vi "TLB Native Dynamic Events ver 0.25.vi"() -> ()   [LabVIEW 2018] (continued)
      tunnel: w233 -> [w2769 w2780 w2794 w2817 w2826 w2840 w2853 w2867 w2881 w2895 w2908 w2919 w2934 w2945 w2967 w2988 w3004 w3012 w3029 w3053 w3063 w3075 w3089 w3101 w3115 w3136 w3171 w3199 w3210 w3222 w3233 w3248 w3263 w3275 w3285 w3311 w3322 w3329 w3339 w3349 w3361 w3373 w3391 w3401 w3417 w3423 w3443 w3457 w3471 w3485 w3499 w3513 w3526]
      tunnel: [w2769 w2780 w2794 w2817 w2826 w2840 w2853 w2867 w2881 w2895 w2908 w2919 w2934 w2945 w2966 w2988 w3004 w3012 w3028 w3053 w3063 w3075 w3089 w3101 w3115 w3135 w3170 w3199 w3210 w3222 w3233 w3248 w3263 w3275 w3285 w3311 w3322 w3329 w3339 w3349 w3361 w3373 w3391 w3401 w3417 w3423 w3443 w3457 w3471 w3485 w3499 w3513 w3526] -> w232
      tunnel: w230 -> [w2767 w2779 w2795 w2818 w2827 w2841 w2854 w2866 w2882 w2896 w2907 w2918 w2933 w2944 w2963 w2989 w3005 w3011 w3025 w3050 w3062 w3074 w3088 w3100 w3114 w3133 w3168 w3197 w3209 w3221 w3232 w3247 w3262 w3274 w3284 w3312 w3323 w3328 w3338 w3348 w3360 w3372 w3392 w3402 w3418 w3422 w3437 w3451 w3465 w3479 w3493 w3507 w3520]
      tunnel: [w2767 w2779 w2795 w2818 w2827 w2841 w2854 w2866 w2882 w2896 w2907 w2918 w2933 w2944 w2963 w2989 w3005 w3011 w3025 w3050 w3062 w3074 w3088 w3100 w3113 w3132 w3167 w3197 w3209 w3221 w3232 w3247 w3262 w3274 w3284 w3312 w3323 w3328 w3338 w3348 w3360 w3372 w3392 w3402 w3418 w3422 w3437 w3449 w3463 w3477 w3491 w3505 w3519] -> w229
      tunnel: w227 -> [_ _ _ _ _ _ _ _ _ _ _ _ _ _ _ _ _ _ _ _ _ _ _ _ _ _ _ _ _ _ _ _ _ _ _ _ _ _ _ _ _ _ _ _ w3409 _ _ _ _ _ _ _ _]
      tunnel: [w2766 w2778 w2789 w2808 w2821 w2835 w2849 w2862 w2877 w2890 w2904 w2917 w2927 w2943 w2960 w2980 w3006 w3010 w3022 w3049 w3061 w3073 w3087 w3097 w3107 w3126 w3159 w3196 w3208 w3220 w3237 w3241 w3256 w3271 w3282 w3296 w3315 w3334 w3337 w3347 w3359 w3371 w3383 w3403 w3407 w3421 w3436 w3446 w3460 w3474 w3488 w3502 w3516] -> w223
      tunnel: w224 -> [w2766 w2778 w2789 w2808 w2821 w2835 w2849 w2862 w2877 w2890 w2904 w2917 w2927 w2943 w2960 w2981 w3006 w3010 w3022 w3049 w3061 w3073 w3087 w3097 w3107 w3127 w3160 w3196 w3208 w3220 w3237 w3241 w3256 w3271 w3282 w3296 w3315 w3334 w3337 w3347 w3359 w3371 w3383 w3403 w3407 w3421 w3436 w3446 w3460 w3474 w3488 w3502 w3516]
      tunnel: w221 -> [_ _ _ _ _ _ _ _ w2876 _ _ _ _ _ _ _ _ _ _ _ _ _ _ _ _ _ _ _ _ _ _ _ _ _ _ _ _ _ _ _ _ _ _ _ _ _ _ _ _ _ _ _ _]
      tunnel: w219 -> [w2765 w2777 w2788 w2802 w2820 w2834 w2848 w2861 w2874 w2889 w2903 w2916 w2926 w2942 w2959 w2976 w2999 w3009 w3020 w3048 w3060 w3072 w3086 w3096 w3110 w3129 w3163 w3195 w3207 w3219 w3229 w3240 w3255 w3270 w3281 w3293 w3314 w3325 w3336 w3346 w3358 w3370 w3382 w3394 w3406 w3420 w3435 w3445 w3459 w3473 w3487 w3501 w3515]
      tunnel: [w2765 w2777 w2788 w2802 w2820 w2834 w2848 w2861 w2874 w2889 w2903 w2916 w2926 w2942 w2959 w2976 w2998 w3009 w3020 w3048 w3060 w3072 w3086 w3096 w3109 w3128 w3162 w3195 w3207 w3219 w3229 w3240 w3255 w3270 w3281 w3293 w3314 w3325 w3336 w3346 w3358 w3370 w3382 w3394 w3406 w3420 w3435 w3445 w3459 w3473 w3487 w3501 w3515] -> w218
      tunnel: [_ _ _ _ _ _ _ _ _ _ _ _ _ _ _ _ _ _ _ _ _ _ _ _ _ _ _ _ _ _ _ _ _ _ _ w3292 _ _ _ _ _ _ _ _ _ _ _ _ _ _ _ _ _] -> w216
      tunnel: w214 -> [w2764 w2776 w2787 w2801 w2819 w2833 w2847 w2860 w2873 w2888 w2902 w2915 w2925 w2941 w2958 w2975 w2990 w3008 w3018 w3047 w3059 w3071 w3085 w3095 w3111 w3130 w3164 w3194 w3206 w3218 w3228 w3239 w3254 w3269 w3280 w3291 w3313 w3324 w3335 w3345 w3357 w3369 w3381 w3393 w3405 w3419 w3434 w3444 w3458 w3472 w3486 w3500 w3514]
      tunnel: [w2764 w2776 w2787 w2801 w2819 w2833 w2847 w2860 w2873 w2888 w2902 w2915 w2925 w2941 w2958 w2975 w2990 w3008 w3018 w3047 w3059 w3071 w3085 w3095 w3111 w3130 w3164 w3194 w3206 w3218 w3228 w3239 w3254 w3269 w3280 w3291 w3313 w3324 w3335 w3345 w3357 w3369 w3381 w3393 w3405 w3419 w3434 w3444 w3458 w3472 w3486 w3500 w3514] -> w213
      frame "Exit" {
        # ">>State Logic  >>"
        # ">>> Time cluster >>>"
        # ">>> Yaw >>>"
        # ">>> Stepper position >>>"
        # ">>> Encoders >>>"
        # ">>> Object detection >>>"
        # ">>> Ultrasonic Sensors Detect >>>"
        n70 = call "Imaq Dispose"("All Images? (No)"=TRUE) -> ()  [unwired: 5 in, 1 out]
      }
      frame "----Movement States----" {
        # ">>State Logic  >>"
        # ">>> Time cluster >>>"
        # ">>> Yaw >>>"
        # ">>> Stepper position >>>"
        # ">>> Encoders >>>"
        # ">>> Object detection >>>"
        # ">>> Ultrasonic Sensors Detect >>>"
      }
      frame "FORWARD" {
        # ">>State Logic  >>"
        # ">>> Time cluster >>>"
        # ">>> Yaw >>>"
        # ">>> Stepper position >>>"
        # ">>> Encoders >>>"
        # ">>> Object detection >>>"
        # ">>> Ultrasonic Sensors Detect >>>"
        n71 = Unbundle By Name(w2794) -> ("Yaw"=w2790:dbl)
        n72 = call "MOTOR CONTROL WITH PID AE.vi"("Yaw"=w2790, "Speed"=50.0, "Direction"=MOTOR_CONTROL_WITH_PID_AE_DIRECTION_TYPE_DEF."y-axis movement", "AE Mode"=MOTOR_CONTROL_WITH_PID_AE_DATA_MODE_TYPE_DEF."Write to AE") -> ()  [unwired: 1 out]
      }
      frame "FORWARD - IR ASSIST" {
        # ">>State Logic  >>"
        # ">>> Time cluster >>>"
        # ">>> Yaw >>>"
        # ">>> Stepper position >>>"
        # ">>> Encoders >>>"
        # ">>> Object detection >>>"
        # ">>> Ultrasonic Sensors Detect >>>"
        n73 = Unbundle By Name(w2808) -> ("Left IR Sensor"=w2807:dbl)
        n74 = Subtract(x=w2807, y=15.0) -> (x-y=w2805:dbl)
        n75 = Multiply(x=w2805, y=0.25) -> (x*y=w2803:dbl)
        n76 = call "MOTOR CONTROL WITH PID AE.vi"("Yaw"=w2803, "Speed"=30.0, "Direction"=MOTOR_CONTROL_WITH_PID_AE_DIRECTION_TYPE_DEF."y-axis movement", "AE Mode"=MOTOR_CONTROL_WITH_PID_AE_DATA_MODE_TYPE_DEF."Write to AE") -> ()  [unwired: 1 out]
      }
      frame "LEFT" {
        # ">>State Logic  >>"
        # ">>> Time cluster >>>"
        # ">>> Yaw >>>"
        # ">>> Stepper position >>>"
        # ">>> Encoders >>>"
        # ">>> Object detection >>>"
        # ">>> Ultrasonic Sensors Detect >>>"
        n77 = Unbundle By Name(w2826) -> ("Yaw"=w2823:dbl)
        n78 = call "MOTOR CONTROL WITH PID AE.vi"("Yaw"=w2823, "Speed"=-20.0, "Direction"=MOTOR_CONTROL_WITH_PID_AE_DIRECTION_TYPE_DEF."x-axis movement", "AE Mode"=MOTOR_CONTROL_WITH_PID_AE_DATA_MODE_TYPE_DEF."Write to AE") -> ()  [unwired: 1 out]
      }
      frame "RIGHT" {
        # ">>> Time cluster >>>"
        # ">>> Yaw >>>"
        # ">>> Stepper position >>>"
        # ">>> Encoders >>>"
        # ">>> Object detection >>>"
        # ">>> Ultrasonic Sensors Detect >>>"
        n79 = Unbundle By Name(w2840) -> ("Yaw"=w2836:dbl)
        n80 = call "MOTOR CONTROL WITH PID AE.vi"("Yaw"=w2836, "Speed"=20.0, "Direction"=MOTOR_CONTROL_WITH_PID_AE_DIRECTION_TYPE_DEF."x-axis movement", "AE Mode"=MOTOR_CONTROL_WITH_PID_AE_DATA_MODE_TYPE_DEF."Write to AE") -> ()  [unwired: 1 out]
      }
      frame "R-ACW" {
        # ">>> IR Sensors >>>"
        # ">>> Time cluster >>>"
        # ">>> Yaw >>>"
        # ">>> Stepper position >>>"
        # ">>> Encoders >>>"
        # ">>> Object detection >>>"
        # ">>> Ultrasonic Sensors Detect >>>"
        n81 = call "MOTOR CONTROL WITH PID AE.vi"("Speed"=10.0, "Direction"=MOTOR_CONTROL_WITH_PID_AE_DIRECTION_TYPE_DEF."rotation", "AE Mode"=MOTOR_CONTROL_WITH_PID_AE_DATA_MODE_TYPE_DEF."Write to AE") -> ()  [unwired: 1 in, 1 out]
      }
      frame "R-CW" {
        (unwired) -0.2 ("Speed")
        # ">>> Time cluster >>>"
        # ">>> Yaw >>>"
        # ">>> Stepper position >>>"
        # ">>> Encoders >>>"
        # ">>> Object detection >>>"
        # ">>> Ultrasonic Sensors Detect >>>"
        n82 = call "MOTOR CONTROL WITH PID AE.vi"("Speed"=-10.0, "Direction"=MOTOR_CONTROL_WITH_PID_AE_DIRECTION_TYPE_DEF."rotation", "AE Mode"=MOTOR_CONTROL_WITH_PID_AE_DATA_MODE_TYPE_DEF."Write to AE") -> ()  [unwired: 1 in, 1 out]
      }
      frame "X AXIS - SLOW" {
        # ">>> Line Sensor Cluster>>>"
        # ">>> IR Sensors >>>"
        # ">>> Time cluster >>>"
        # ">>> Yaw >>>"
        # ">>> Stepper position >>>"
        # ">>> Encoders >>>"
        # ">>> Object detection >>>"
        # ">>> Ultrasonic Sensors Detect >>>"
        n83 = Unbundle By Name(w2876) -> ("xSpeed"=w2875:dbl)
        n84 = Unbundle By Name(w2881) -> ("Yaw"=w2878:dbl)
        n85 = call "MOTOR CONTROL WITH PID AE.vi"("Yaw"=w2878, "Speed"=w2875, "Direction"=MOTOR_CONTROL_WITH_PID_AE_DIRECTION_TYPE_DEF."x-axis movement", "AE Mode"=MOTOR_CONTROL_WITH_PID_AE_DATA_MODE_TYPE_DEF."Write to AE") -> ()  [unwired: 1 out]
      }
      frame "REVERSE" {
        # ">>> Time cluster >>>"
        # ">>> Yaw >>>"
        # ">>> Stepper position >>>"
        # ">>> Encoders >>>"
        # ">>> Object detection >>>"
        # ">>> Ultrasonic Sensors Detect >>>"
        n86 = Unbundle By Name(w2895) -> ("Yaw"=w2891:dbl)
        n87 = call "MOTOR CONTROL WITH PID AE.vi"("Yaw"=w2891, "Speed"=-50.0, "Direction"=MOTOR_CONTROL_WITH_PID_AE_DIRECTION_TYPE_DEF."y-axis movement", "AE Mode"=MOTOR_CONTROL_WITH_PID_AE_DATA_MODE_TYPE_DEF."Write to AE") -> ()  [unwired: 1 out]
      }
      frame "STOP" {
        n88 = Wait (ms)(milliseconds to wait=u32 100) -> ()  [unwired: 1 out]
        n89 = call "MOTOR CONTROL WITH PID AE.vi"("Direction"=MOTOR_CONTROL_WITH_PID_AE_DIRECTION_TYPE_DEF."stop", "AE Mode"=MOTOR_CONTROL_WITH_PID_AE_DATA_MODE_TYPE_DEF."Write to AE") -> ()  [unwired: 2 in, 1 out]
      }
      frame "----SENSOR READING---- " {
      }
      frame "READ ENCODERS" {
        # ">>> Time cluster >>>"
        # ">>> Yaw >>>"
        # ">>> Stepper position >>>"
        # ">>> Object detection >>>"
        # ">>> Current encoder distance >>>"
        # ">>> Ultrasonic Sensors Detect >>>"
        n90 = call "MOTOR CONTROL WITH PID AE.vi"("AE Mode"=MOTOR_CONTROL_WITH_PID_AE_DATA_MODE_TYPE_DEF."Read from AE") -> ("Speed & distance"=w2931:T13)  [unwired: 3 in]
        n91 = Unbundle By Name(w2931) -> ("xDistance"=w2930:dbl, "yDistance"=w2929:dbl, "wDistance"=w2928:dbl)
        n92 = Bundle By Name(cluster=w2938, "xDistance"=w2930, "yDistance"=w2929, "wDistance"=w2928) -> (w2937:T6)
      }
      frame "READ ULTRASONIC" {
        (unwired) navX_type_def."Read Values" ("Mode")
        (unwired) MOTOR_CONTROL_NO_PID_Type_Def."Latch" ("Direction")
        # ">>> Line Sensor Cluster>>>"
        # ">>> IR Sensors >>>"
        # ">>State Logic  >>"
        # ">>> Time cluster >>>"
        # ">>> Ultrasonic Sensors Detect >>>"
        # ">>> Object detection >>>"
        # ">>> Encoders >>>"
        # ">>> Stepper position >>>"
        # ">>> Yaw >>>"
        n93 = call "Arduino Interfacing VI.vi"("AE Mode"=Arduino_Interfacing."Read From Arduino") -> ("Arduino Data"=w2950:T15)  [unwired: 3 in, 1 out]
        n94 = Unbundle By Name(w2950) -> ("PING A"=w2949:u8, "PING B"=w2948:u8, "PING C"=w2947:u8, "PING D"=w2946:u8)
        n95 = Bundle By Name(cluster=w2956, "PING_A"=w2949, "PING_B"=w2948, "PING_C"=w2947, "PING_D"=w2946) -> (w2957:T7)
      }
      frame "READ NAVX" {
        # ">> Item Selection Bias >>"
        # ">>State Logic  >>"
        # ">>> Line Sensor Cluster>>>"
        # ">>> IR Sensors >>>"
        # ">>> Time cluster >>>"
        # ">>> Yaw >>>"
        # ">>> Ultrasonic Sensors Detect >>>"
        # ">>> Object detection >>>"
        # ">>> Encoders >>>"
        # ">>> Stepper position >>>"
        n96 = call "navX reading VI.vi"("Mode"=navX_type_def."Read Values") -> ("NavX Readings"=w2962:T14)  [unwired: 2 in, 3 out]
        n97 = Unbundle By Name(w2962) -> ("Heading"=w2961:dbl)
        n98 = Unbundle By Name(w2962) -> ("Yaw"=w2965:dbl)
        n99 = Bundle By Name(cluster=w2967, "Yaw"=w2965, "Compass"=w2961) -> (w2966:T4)
      }
      frame "READ IR" {
        w2974 = T38 [enum."B/AI2"] items=["Not Connected", "AudioIn/Left", "AudioIn/Right", "C/AI0", "C/AI1", "A/AI0", "A/AI1", "A/AI2", "A/AI3", "A/AI4", "A/AI5", "A/AI6", "A/AI7", "B/AI0", "B/AI1", "B/AI2", "B/AI3", "B/AI4", "B/AI5", "B/AI6", "B/AI7", "AI/AI0", "AI/AI1", "AI/AI2", "AI/AI3", "A/AI0 (DIFF)", "A/AI1 (DIFF)", "A/AI2 (DIFF)", "A/AI3 (DIFF)", "B/AI0 (DIFF)", "B/AI1 (DIFF)", "B/AI2 (DIFF)", "B/AI3 (DIFF)"] ("AI Channel")
        w2978 = T38 [enum."B/AI1"] items=["Not Connected", "AudioIn/Left", "AudioIn/Right", "C/AI0", "C/AI1", "A/AI0", "A/AI1", "A/AI2", "A/AI3", "A/AI4", "A/AI5", "A/AI6", "A/AI7", "B/AI0", "B/AI1", "B/AI2", "B/AI3", "B/AI4", "B/AI5", "B/AI6", "B/AI7", "AI/AI0", "AI/AI1", "AI/AI2", "AI/AI3", "A/AI0 (DIFF)", "A/AI1 (DIFF)", "A/AI2 (DIFF)", "A/AI3 (DIFF)", "B/AI0 (DIFF)", "B/AI1 (DIFF)", "B/AI2 (DIFF)", "B/AI3 (DIFF)"] ("AI Channel")
        w2983 = T38 [enum."B/AI0"] items=["Not Connected", "AudioIn/Left", "AudioIn/Right", "C/AI0", "C/AI1", "A/AI0", "A/AI1", "A/AI2", "A/AI3", "A/AI4", "A/AI5", "A/AI6", "A/AI7", "B/AI0", "B/AI1", "B/AI2", "B/AI3", "B/AI4", "B/AI5", "B/AI6", "B/AI7", "AI/AI0", "AI/AI1", "AI/AI2", "AI/AI3", "A/AI0 (DIFF)", "A/AI1 (DIFF)", "A/AI2 (DIFF)", "A/AI3 (DIFF)", "B/AI0 (DIFF)", "B/AI1 (DIFF)", "B/AI2 (DIFF)", "B/AI3 (DIFF)"] ("AI Channel")
        # ">>> Line Sensor Cluster>>>"
        # ">>> IR Sensors >>>"
        # ">>State Logic  >>"
        # ">>> Time cluster >>>"
        # ">>> Ultrasonic Sensors Detect >>>"
        # ">>> Object detection >>>"
        # ">>> Encoders >>>"
        # ">>> Stepper position >>>"
        # ">>> Yaw >>>"
        n100 = call <vilib>:"Sharp IR.vi"("AI Channel"=w2983) -> ("Sharp IR Distance"=w2979:dbl)  [unwired: 8 in, 2 out]
        n101 = call <vilib>:"Sharp IR.vi"("AI Channel"=w2978) -> ("Sharp IR Distance"=w2977:dbl)  [unwired: 8 in, 2 out]
        n102 = call <vilib>:"Sharp IR.vi"("AI Channel"=w2974) -> ("Sharp IR Distance"=w2973:dbl)  [unwired: 8 in, 2 out]
        n103 = Bundle By Name(cluster=w2981, "Left IR Sensor"=w2979, "Arm IR Sensor"=w2977, "Bottom IR Sensor"=w2973) -> (w2980:T3)
      }
      frame "READ LINE SENSOR" {
        # ">>> IR Sensors >>>"
        # ">>> Line Sensor Cluster>>>"
        # ">>State Logic  >>"
        # ">>> Time cluster >>>"
        # ">>> Object detection >>>"
        # ">>> Yaw >>>"
        # ">>> Ultrasonic Sensors Detect >>>"
        # ">>> Encoders >>>"
        # ">>> Stepper position >>>"
        n104 = call "Line Sensor AE.vi"("AE State"=Line_Sensor_AE_Type_Def."READ FROM LINE SENSORS") -> ("Line Detected?"=w2996:bool, "Line Sensor Raw Values"=w2995:T40)
        n105 = Unbundle By Name(w2995) -> ("S1"=w2994:dbl, "S2"=w2993:dbl, "S3"=w2992:dbl, "S4"=w2991:dbl)
        n106 = Bundle By Name(cluster=w2999, "Line Detected?"=w2996, "S1"=w2994, "S2"=w2993, "S3"=w2992, "S4"=w2991) -> (w2998:T2)
      }
      frame "----SYSTEM MODES----" {
        (unwired) I2C_MASTER_Type_Def."Last State" ("Arduino Mode")
        # ">>> Object detection >>>"
        # ">>> Yaw >>>"
        # ">>> Ultrasonic Sensors Detect >>>"
        # ">>> Encoders >>>"
        # ">>> Stepper position >>>"
      }
      frame "INIT" {
        w3040 = u8 0
        w3041 = 0.0
        # ">>> IR Sensors >>>"
        # ">>> IR Sensors >>>"
        # ">>> Line Sensor Cluster>>>"
        # ">>> Time cluster >>>"
        # ">>> Object detection >>>"
        # ">>> Yaw >>>"
        # ">>> Ultrasonic Sensors Detect >>>"
        # ">>> Encoders >>>"
        # ">>> Stepper position >>>"
        # ">>State Logic  >>"
        n107 = call "Arduino Interfacing VI.vi"("AE Mode"=Arduino_Interfacing."Initialize") -> ()  [unwired: 3 in, 2 out]
        n108 = call "FGV Stop.vi"("Init/Read/Write State"=States_for_Action_Engine."Initialize") -> ()  [unwired: 2 in, 2 out]
        n109 = call "Elasped Timer.vi"("Action"=Elapsed_timer_control."Initialize") -> ()  [unwired: 7 in, 4 out]
        n110 = call "MOTOR CONTROL WITH PID AE.vi"("AE Mode"=MOTOR_CONTROL_WITH_PID_AE_DATA_MODE_TYPE_DEF."Init AE") -> ()  [unwired: 3 in, 1 out]
        n111 = call "IMAQ Reference AE.vi"("IMAQ AE States"=IMAQ_Reference_AE."Initialize AE") -> ()  [unwired: 1 in, 2 out]
        n112 = call "Line Sensor AE.vi"("AE State"=Line_Sensor_AE_Type_Def."INIT AE") -> ()  [unwired: 2 out]
        n113 = Bundle By Name(cluster=w3034, "Recognized Object"=FALSE, "Object X coordinate"=0.0, "Object Y coordinate"=0.0) -> (w3033:T9)
        n114 = Bundle By Name(cluster=w3039, "y Stepper Position"=u8 0, "z Stepper Position"=u8 0) -> (w3038:T5)
        n115 = Bundle By Name(cluster=w3043, "xDistance"=w3041, "yDistance"=w3041, "wDistance"=w3041) -> (w3042:T6)
        n116 = Bundle By Name(cluster=w3045, "PING_A"=w3040, "PING_B"=w3040, "PING_C"=w3040, "PING_D"=w3040) -> (w3046:T7)
        n117 = Bundle By Name(cluster=w3029, "Yaw"=0.0) -> (w3028:T4)
      }
      frame "ARDUINO - ULTRASONIC" {
        # ">>> Time cluster >>>"
        # ">>> Line Sensor Cluster>>>"
        # ">>> Object detection >>>"
        # ">>> Yaw >>>"
        # ">>> Ultrasonic Sensors Detect >>>"
        # ">>> Encoders >>>"
        # ">>> Stepper position >>>"
        # ">>State Logic  >>"
        n118 = call "Arduino Interfacing VI.vi"("Data to Write"=I2C_MASTER_WRITE_NEW_Type_Def."Ultrasonic sensors", "AE Mode"=Arduino_Interfacing."Write to Arduino") -> ()  [unwired: 2 in, 2 out]
      }
      frame "NAVX CALIBRATE" {
        # ">>> Object detection >>>"
        # ">>> Yaw >>>"
        # ">>> Ultrasonic Sensors Detect >>>"
        # ">>> Encoders >>>"
        # ">>> Stepper position >>>"
        # ">>State Logic  >>"
        # "Adds a 15 second delay to the startup process \nfor the NavX to calibrate"
        n119 = Wait (ms)(milliseconds to wait=u32 1000) -> ()  [unwired: 1 out]
      }
      frame "NO ACTION", Default {
        (unwired) u8 0 ("y Stepper value")
        (unwired) TRUE ("Latch")
        (unwired) navX_type_def."Read Values" ("Mode")
        (unwired) MOTOR_CONTROL_NO_PID_Type_Def."Latch" ("Direction")
        # ">>> Object detection >>>"
        # ">>> Yaw >>>"
        # ">>> Ultrasonic Sensors Detect >>>"
        # ">>> Encoders >>>"
        # ">>> Stepper position >>>"
        # ">>State Logic  >>"
        n120 = case shown="4" w3079 {
          tunnel: [0 100] -> w3081
          frame 1, Default {
          }
          frame 4 {
          }
        }
      }
      frame "----RESET CASES----" {
        (unwired) I2C_MASTER_Type_Def."Last State" ("Arduino Mode")
        # ">>> Object detection >>>"
        # ">>> Yaw >>>"
        # ">>> Ultrasonic Sensors Detect >>>"
        # ">>> Encoders >>>"
        # ">>> Stepper position >>>"
        # ">>State Logic  >>"
      }
      frame "RESET ENCODERS" {
        # ">>> Object detection >>>"
        # ">>> Yaw >>>"
        # ">>> Ultrasonic Sensors Detect >>>"
        # ">>> Encoders >>>"
        # ">>> Stepper position >>>"
        # ">>State Logic  >>"
        n121 = call "MOTOR CONTROL WITH PID AE.vi"("Direction"=MOTOR_CONTROL_WITH_PID_AE_DIRECTION_TYPE_DEF."reset encoders", "AE Mode"=MOTOR_CONTROL_WITH_PID_AE_DATA_MODE_TYPE_DEF."Write to AE") -> ()  [unwired: 2 in, 1 out]
      }
      frame "RESET FLAGS" {
        # ">>> Line Sensor Cluster>>>"
        # ">>> IR Sensors >>>"
        # ">>> Time cluster >>>"
        # ">>> Object detection >>>"
        # ">>> Yaw >>>"
        # ">>> Ultrasonic Sensors Detect >>>"
        # ">>> Encoders >>>"
        # ">>> Stepper position >>>"
        # ">>> Line Sensor Cluster>>>"
        # ">>> IR Sensors >>>"
        # ">>> Time cluster >>>"
        # ">>> Object detection >>>"
        # ">>> Yaw >>>"
        # ">>> Ultrasonic Sensors Detect >>>"
        # ">>> Encoders >>>"
        # ">>> Stepper position >>>"
        # "Resets BOOLEAN FLAGS only"
        n122 = Wait (ms)(milliseconds to wait=u32 20) -> ()  [unwired: 1 out]
        n123 = Bundle By Name(cluster=w3120, "Recognized Object"=FALSE) -> (w3119:T9)
        n124 = Bundle By Name(cluster=w3110, "Line Detected?"=FALSE) -> (w3109:T2)
        n125 = Bundle By Name(cluster=w3114, "Time up flag"=FALSE) -> (w3113:T1)
      }
      frame "RESET SENSOR VALUES" {
        w3124 = 0.0 ("S4")
        w3125 = 0.0 ("S4")
        # "Resets SENSOR VALUES only"
        # ">>> Line Sensor Cluster>>>"
        # ">>> IR Sensors >>>"
        # ">>> Time cluster >>>"
        # ">>> Object detection >>>"
        # ">>> Yaw >>>"
        # ">>> Ultrasonic Sensors Detect >>>"
        # ">>> Encoders >>>"
        # ">>> Stepper position >>>"
        # ">>> Line Sensor Cluster>>>"
        # ">>> IR Sensors >>>"
        # ">>> Time cluster >>>"
        # ">>> Object detection >>>"
        # ">>> Yaw >>>"
        # ">>> Ultrasonic Sensors Detect >>>"
        # ">>> Encoders >>>"
        # ">>> Stepper position >>>"
        # "Resets any software variables\nand/or non-critical states"
        n126 = Wait (ms)(milliseconds to wait=u32 20) -> ()  [unwired: 1 out]
        n127 = Bundle By Name(cluster=w3133, "SET TIME TO CHECK"=0.0) -> (w3132:T1)
        n128 = Bundle By Name(cluster=w3149, "Object X coordinate"=0.0, "Object Y coordinate"=0.0) -> (w3148:T9)
        n129 = Bundle By Name(cluster=w3140, "y Stepper Position"=u8 0, "z Stepper Position"=u8 0) -> (w3139:T5)
        n130 = Bundle By Name(cluster=w3127, "Left IR Sensor"=w3124, "Arm IR Sensor"=w3124) -> (w3126:T3)
        n131 = Bundle By Name(cluster=w3145, "xDistance"=0.0, "yDistance"=0.0, "wDistance"=0.0) -> (w3144:T6)
        n132 = Bundle By Name(cluster=w3156, "PING_A"=u8 0, "PING_B"=u8 0, "PING_C"=u8 0, "PING_D"=u8 0) -> (w3155:T7)
        n133 = Bundle By Name(cluster=w3136, "Yaw"=0.0) -> (w3135:T4)
        n134 = Bundle By Name(cluster=w3129, "S1"=w3125, "S2"=w3125, "S3"=w3125, "S4"=w3125) -> (w3128:T2)
      }
      frame "RESET ALL SENSORS" {
        w3158 = 0.0 ("SET TIME TO CHECK")
        # ">>> Line Sensor Cluster>>>"
        # ">>> IR Sensors >>>"
        # ">>> Time cluster >>>"
        # ">>> Object detection >>>"
        # ">>> Yaw >>>"
        # ">>> Ultrasonic Sensors Detect >>>"
        # ">>> Encoders >>>"
        # ">>> Stepper position >>>"
        # ">>> Line Sensor Cluster>>>"
        # ">>> IR Sensors >>>"
        # ">>> Time cluster >>>"
        # ">>> Object detection >>>"
        # ">>> Yaw >>>"
        # ">>> Ultrasonic Sensors Detect >>>"
        # ">>> Encoders >>>"
        # ">>> Stepper position >>>"
        # "Resets ALL SENSOR PARAMTERS"
        n135 = Wait (ms)(milliseconds to wait=u32 20) -> ()  [unwired: 1 out]
        n136 = Bundle By Name(cluster=w3168, "Time up flag"=FALSE, "SET TIME TO CHECK"=0.0) -> (w3167:T1)
        n137 = Bundle By Name(cluster=w3185, "Recognized Object"=FALSE, "Object X coordinate"=0.0, "Object Y coordinate"=0.0) -> (w3184:T9)
        n138 = Bundle By Name(cluster=w3175, "y Stepper Position"=u8 0, "z Stepper Position"=u8 0) -> (w3174:T5)
        n139 = Bundle By Name(cluster=w3163, "Line Detected?"=FALSE) -> (w3162:T2)
        n140 = Bundle By Name(cluster=w3160, "Left IR Sensor"=w3158, "Arm IR Sensor"=w3158) -> (w3159:T3)
        n141 = Bundle By Name(cluster=w3180, "xDistance"=0.0, "yDistance"=0.0, "wDistance"=0.0) -> (w3179:T6)
        n142 = Bundle By Name(cluster=w3192, "PING_A"=u8 0, "PING_B"=u8 0, "PING_C"=u8 0, "PING_D"=u8 0) -> (w3191:T7)
        n143 = Bundle By Name(cluster=w3171, "Yaw"=0.0) -> (w3170:T4)
      }
      frame "RESET YAW" {
        n144 = Wait (ms)(milliseconds to wait=u32 100) -> ()  [unwired: 1 out]
        n145 = call "navX reading VI.vi"("Mode"=navX_type_def."Zero Yaw") -> ()  [unwired: 2 in, 4 out]
      }
      frame "RESET ARM" {
        n146 = call "Arduino Interfacing VI.vi"("Data to Write"=I2C_MASTER_WRITE_NEW_Type_Def."Soft Reset", "AE Mode"=Arduino_Interfacing."Write to Arduino") -> ()  [unwired: 2 in, 2 out]
      }
      frame "--------CAM STATES-------" {
      }
      frame "OPEN IMAQ REF" {
        # ">>> Line Sensor Cluster>>>"
        # ">>State Logic  >>"
        # ">>> Time cluster >>>"
        # ">>> Object detection >>>"
        # ">>> Yaw >>>"
        # ">>> Ultrasonic Sensors Detect >>>"
        # ">>> Encoders >>>"
        # ">>> Stepper position >>>"
        # ">>> IR Sensors >>>"
        n147 = call "IMAQ Reference AE.vi"("IMAQ AE States"=IMAQ_Reference_AE."Initialize AE") -> ()  [unwired: 1 in, 2 out]
      }
      frame "OPEN LOG CAM" {
        n148 = call "Webcam AE.vi"("Session In"=T36 "cam0", "Camera states"=Webcam_AE."Initialize Camera") -> ("error out"=w3244:errorcluster, "Session Out"=w3243:T36)  [unwired: 1 in, 1 out]
        n149 = call "Webcam AE.vi"("error in (no error)"=w3244, "Session In"=w3243, "Camera states"=Webcam_AE."Open Camera") -> ()  [unwired: 3 out]
      }
      frame "OPEN LIFE CAM" {
        n150 = call "Webcam AE.vi"("Session In"=T36 "cam1", "Camera states"=Webcam_AE."Initialize Camera") -> ("error out"=w3259:errorcluster, "Session Out"=w3258:T36)  [unwired: 1 in, 1 out]
        n151 = call "Webcam AE.vi"("error in (no error)"=w3259, "Session In"=w3258, "Camera states"=Webcam_AE."Open Camera") -> ()  [unwired: 3 out]
      }
      frame "CAM ACQ" {
        # ">>State Logic  >>"
        # ">>> Time cluster >>>"
        # ">>> Yaw >>>"
        # ">>> Stepper position >>>"
        # ">>> Encoders >>>"
        # ">>> Object detection >>>"
        # ">>> Ultrasonic Sensors Detect >>>"
        n152 = call "Webcam AE.vi"("Camera states"=Webcam_AE."Continuous Acquisition") -> ()  [unwired: 2 in, 3 out]
      }
      frame "CAM CLOSE" {
        # ">>State Logic  >>"
        # ">>> Time cluster >>>"
        # ">>> Yaw >>>"
        # ">>> Stepper position >>>"
        # ">>> Encoders >>>"
        # ">>> Object detection >>>"
        # ">>> Ultrasonic Sensors Detect >>>"
        n153 = call "Webcam AE.vi"("Camera states"=Webcam_AE."Close Camera") -> ()  [unwired: 2 in, 3 out]
      }
      frame "PROCESS IMAGE" {
        # ">>> Line Sensor Cluster>>>"
        # ">>> IR Sensors >>>"
        # ">> Item Selection Bias >>"
        # ">> Item Selection Bias >>"
        # ">>State Logic  >>"
        # ">>> Time cluster >>>"
        # ">>> Yaw >>>"
        # ">>> Stepper position >>>"
        # ">>> Encoders >>>"
        # ">>> Object detection >>>"
        # ">>> Ultrasonic Sensors Detect >>>"
        n154 = call "Webcam AE.vi"("Camera states"=Webcam_AE."Retrieve Image") -> ("error out"=w3304:errorcluster, "Image Out"=w3305:T42)  [unwired: 2 in, 1 out]
        n155 = call "IMAQ Reference AE.vi"("IMAQ AE States"=IMAQ_Reference_AE."Get IMAQ Reference") -> ("Image Out"=w3294:T42)  [unwired: 1 in, 1 out]
        n156 = call "Object Detection SubVI.vi"("Error In"=w3304, "Mode"=w3291, "Image Dest"=w3294, "Image in"=w3305) -> ("Error out"=w3292:errorcluster, "Object Center Coordinates"=w3301:cluster{"x":sgl, "y":sgl}, "Object detection cluster"=w3297:T43)  [unwired: 1 out]
        n157 = Unbundle By Name(w3297) -> ("Object detected?"=w3298:bool)
        n158 = Unbundle By Name(w3301) -> ("x"=w3300:sgl, "y"=w3299:sgl)
        n159 = Bundle By Name(cluster=w3303, "Recognized Object"=w3298, "Object X coordinate"=w3300, "Object Y coordinate"=w3299) -> (w3302:T9)
      }
      frame "DISPOSE CAM BUFFERS" {
        # ">> Item Selection Bias >>"
        # ">>> Line Sensor Cluster>>>"
        # ">>> IR Sensors >>>"
        # ">>State Logic  >>"
        # ">>> Time cluster >>>"
        # ">>> Yaw >>>"
        # ">>> Stepper position >>>"
        # ">>> Encoders >>>"
        # ">>> Object detection >>>"
        # ">>> Ultrasonic Sensors Detect >>>"
        n160 = call "Webcam AE.vi"("Camera states"=Webcam_AE."Dispose Camera Image Buffer") -> ()  [unwired: 2 in, 3 out]
      }
      frame "DISPOSE PROC BUFFERS" {
        # ">>> Line Sensor Cluster>>>"
        # ">>State Logic  >>"
        # ">>> IR Sensors >>>"
        # ">>> Time cluster >>>"
        # ">>> Object detection >>>"
        # ">>> Yaw >>>"
        # ">>> Ultrasonic Sensors Detect >>>"
        # ">>> Encoders >>>"
        # ">>> Stepper position >>>"
        n161 = call "IMAQ Reference AE.vi"("IMAQ AE States"=IMAQ_Reference_AE."Dispose Processing Buffer") -> ()  [unwired: 1 in, 2 out]
      }
      frame "-----ARM ACTIONS-----" {
      }
      frame "CLOSE CLAW" {
        n162 = call "Arduino Interfacing VI.vi"("Data to Write"=I2C_MASTER_WRITE_NEW_Type_Def."Close Claw", "AE Mode"=Arduino_Interfacing."Write to Arduino") -> ()  [unwired: 2 in, 2 out]
      }
      frame "OPEN CLAW" {
        n163 = call "Arduino Interfacing VI.vi"("Data to Write"=I2C_MASTER_WRITE_NEW_Type_Def."Open Claw", "AE Mode"=Arduino_Interfacing."Write to Arduino") -> ()  [unwired: 2 in, 2 out]
      }
      frame "Z STEPPER CAM HEIGHT" {
        n164 = call "Arduino Interfacing VI.vi"("Data to Write"=I2C_MASTER_WRITE_NEW_Type_Def."zStepper 6k", "AE Mode"=Arduino_Interfacing."Write to Arduino") -> ()  [unwired: 2 in, 2 out]
      }
      frame "Z STEPPER GRAB HEIGHT" {
        # ">>State Logic  >>"
        # ">>> Time cluster >>>"
        # ">>> Yaw >>>"
        # ">>> Stepper position >>>"
        # ">>> Encoders >>>"
        # ">>> Object detection >>>"
        # ">>> Ultrasonic Sensors Detect >>>"
        n165 = call "Arduino Interfacing VI.vi"("Data to Write"=I2C_MASTER_WRITE_NEW_Type_Def."zStepper 100", "AE Mode"=Arduino_Interfacing."Write to Arduino") -> ()  [unwired: 2 in, 2 out]
      }
      frame "Z STEPPER BOX HEIGHT" {
        # ">>> IR Sensors >>>"
        # ">>> Time cluster >>>"
        # ">>> Yaw >>>"
        # ">>> Stepper position >>>"
        # ">>> Encoders >>>"
        # ">>> Object detection >>>"
        # ">>> Ultrasonic Sensors Detect >>>"
        n166 = call "Arduino Interfacing VI.vi"("Data to Write"=I2C_MASTER_WRITE_NEW_Type_Def."zStepper 4k", "AE Mode"=Arduino_Interfacing."Write to Arduino") -> ()  [unwired: 2 in, 2 out]
      }
      frame "Y STEPPER CONTROL" {
        # ">>State Logic  >>"
        # ">>> yStepper command>>>"
        # ">>> Time cluster >>>"
        # ">>> Yaw >>>"
        # ">>> Stepper position >>>"
        # ">>> Encoders >>>"
        # ">>> Object detection >>>"
        # ">>> Ultrasonic Sensors Detect >>>"
        n167 = Unbundle By Name(w3409) -> ("yStepper desired"=w3408:u8)
        n168 = call "Arduino Interfacing VI.vi"("y Stepper value"=w3408, "Data to Write"=I2C_MASTER_WRITE_NEW_Type_Def."yStepper control", "AE Mode"=Arduino_Interfacing."Write to Arduino") -> ()  [unwired: 1 in, 2 out]
      }
      frame "READ STEPPER VALUES" {
        # ">>State Logic  >>"
        # ">>> Time cluster >>>"
        # ">>> Yaw >>>"
        # ">>> Stepper position >>>"
        # ">>> Encoders >>>"
        # ">>> Object detection >>>"
        # ">>> Ultrasonic Sensors Detect >>>"
        n169 = call "Arduino Interfacing VI.vi"("AE Mode"=Arduino_Interfacing."Read From Arduino") -> ("Arduino Data"=w3426:T15)  [unwired: 3 in, 1 out]
        n170 = Unbundle By Name(w3426) -> ("y Stepper Position"=w3425:u8, "z Stepper Position"=w3424:u8)
        n171 = Bundle By Name(cluster=w3429, "y Stepper Position"=w3425, "z Stepper Position"=w3424) -> (w3428:T5)
      }
      frame " -----TIMING-----" {
        # ">>State Logic  >>"
        # ">>> Time cluster >>>"
        # ">>> Yaw >>>"
        # ">>> Stepper position >>>"
        # ">>> Encoders >>>"
        # ">>> Object detection >>>"
        # ">>> Ultrasonic Sensors Detect >>>"
      }
      frame "SET TIMER 1" {
        # ">>State Logic  >>"
        # ">>> Time cluster >>>"
        # ">>> Yaw >>>"
        # ">>> Stepper position >>>"
        # ">>> Encoders >>>"
        # ">>> Object detection >>>"
        # ">>> Ultrasonic Sensors Detect >>>"
        n172 = call "Elasped Timer.vi"("Time Setting"=1.0, "Action"=Elapsed_timer_control."Initialize") -> ()  [unwired: 6 in, 4 out]
        n173 = Bundle By Name(cluster=w3451, "Time up flag"=FALSE) -> (w3449:T1)
      }
      frame "SET TIMER 2" {
        # ">>State Logic  >>"
        # ">>> Time cluster >>>"
        # ">>> Yaw >>>"
        # ">>> Stepper position >>>"
        # ">>> Encoders >>>"
        # ">>> Object detection >>>"
        # ">>> Ultrasonic Sensors Detect >>>"
        n174 = call "Elasped Timer.vi"("Time Setting"=2.0, "Action"=Elapsed_timer_control."Initialize") -> ()  [unwired: 6 in, 4 out]
        n175 = Bundle By Name(cluster=w3465, "Time up flag"=FALSE) -> (w3463:T1)
      }
      frame "SET TIMER 3" {
        # ">>State Logic  >>"
        # ">>> Time cluster >>>"
        # ">>> Yaw >>>"
        # ">>> Stepper position >>>"
        # ">>> Encoders >>>"
        # ">>> Object detection >>>"
        # ">>> Ultrasonic Sensors Detect >>>"
        n176 = call "Elasped Timer.vi"("Time Setting"=3.0, "Action"=Elapsed_timer_control."Initialize") -> ()  [unwired: 6 in, 4 out]
        n177 = Bundle By Name(cluster=w3479, "Time up flag"=FALSE) -> (w3477:T1)
      }
      frame "SET TIMER 4" {
        # ">>State Logic  >>"
        # ">>> Time cluster >>>"
        # ">>> Yaw >>>"
        # ">>> Stepper position >>>"
        # ">>> Encoders >>>"
        # ">>> Object detection >>>"
        # ">>> Ultrasonic Sensors Detect >>>"
        n178 = call "Elasped Timer.vi"("Time Setting"=4.0, "Action"=Elapsed_timer_control."Initialize") -> ()  [unwired: 6 in, 4 out]
        n179 = Bundle By Name(cluster=w3493, "Time up flag"=FALSE) -> (w3491:T1)
      }
      frame "SET TIMER 5" {
        # ">>State Logic  >>"
        # ">>> Time cluster >>>"
        # ">>> Yaw >>>"
        # ">>> Stepper position >>>"
        # ">>> Encoders >>>"
        # ">>> Object detection >>>"
        # ">>> Ultrasonic Sensors Detect >>>"
        n180 = call "Elasped Timer.vi"("Time Setting"=5.0, "Action"=Elapsed_timer_control."Initialize") -> ()  [unwired: 6 in, 4 out]
        n181 = Bundle By Name(cluster=w3507, "Time up flag"=FALSE) -> (w3505:T1)
      }
      frame "START TIMER" {
        # ">>State Logic  >>"
        # ">>> Time cluster >>>"
        # ">>> Yaw >>>"
        # ">>> Stepper position >>>"
        # ">>> Encoders >>>"
        # ">>> Object detection >>>"
        # ">>> Ultrasonic Sensors Detect >>>"
        n182 = call "Elasped Timer.vi"("Action"=Elapsed_timer_control."Start") -> ("Time Out?!"=w3517:bool)  [unwired: 7 in, 3 out]
        n183 = Bundle By Name(cluster=w3520, "Time up flag"=w3517) -> (w3519:T1)
      }
    }
    "State Logic" <- w249
    "Image Processing Error" <- w216
    n184 = local read "TASK ENABLE"() -> (w243:bool)
    n185 = Not(x=w243) -> (.not. x?=w242:bool)
    n186 = case shown="True" w250 {
      tunnel: w254 -> [w281 w325]
      tunnel: w258 -> [w277 w327]
      tunnel: [w281 w325] -> w263
      tunnel: [w277 w328] -> w262
      tunnel: w259 -> [_ w323]
      tunnel: w261 -> [_ w324]
      tunnel: w256 -> [w280 w330]
      tunnel: [w280 w330] -> w255
      tunnel: "STOP TASK" -> [_ w313]
      tunnel: w249 -> [w279 w329]
      tunnel: [w279 w326] -> w248
      tunnel: w245 -> [w278 w319]
      tunnel: [w278 w319] -> w244
      tunnel: w242 -> [_ w314]
      tunnel: [w276 w311] -> w241
      tunnel: w240 -> [w276 w310]
      tunnel: w238 -> [w275 w307]
      tunnel: [w275 w307] -> w237
      tunnel: w235 -> [w274 w303]
      tunnel: [w274 w303] -> w234
      tunnel: w232 -> [w273 w301]
      tunnel: [w273 w301] -> w231
      tunnel: w229 -> [w272 w299]
      tunnel: [w272 w299] -> w228
      tunnel: w227 -> [w271 w298]
      tunnel: [w271 w297] -> w226
      tunnel: [_ w295] -> w225
      tunnel: w223 -> [w270 w293]
      tunnel: [w270 w293] -> w222
      tunnel: w221 -> [w269 w292]
      tunnel: [w269 w291] -> w220
      tunnel: w218 -> [w268 w288]
      tunnel: [w268 w288] -> w217
      tunnel: [w267 w287] -> w215
      tunnel: w213 -> [w267 w286]
      tunnel: [_ w284] -> w212
      tunnel: [_ w283] -> w211
      tunnel: [_ w282] -> w210
      frame False {
        # ">> Item Selection Bias >>"
        # ">>State Logic Queue Reference >>"
        # ">>Action states Queue Reference >>"
        # ">>True Stop Next State >>"
        # ">>State Logic  >>"
        # ">>> IR Sensors >>>"
        # ">>> Line Sensor Cluster>>>"
        # ">>> Line Sensor Cluster>>>"
        # ">>> Motor control cluster >>>"
        # ">>> yStepper command>>>"
        # ">>> Motor control cluster >>>"
        # ">>> yStepper command>>>"
        # ">>> Motor control cluster >>>"
        # ">>> IR Sensors >>>"
        # ">>> IR Sensors >>>"
        # ">>> yStepper command>>>"
        # ">>> Time cluster >>>"
        # ">>> Yaw >>>"
        # ">>> Stepper position >>>"
        # ">>> Encoders >>>"
        # ">>> Object detection >>>"
        # ">>> Ultrasonic Sensors Detect >>>"
        # ">>> Time cluster >>>"
        # ">>> Yaw >>>"
        # ">>> Stepper position >>>"
        # ">>> Encoders >>>"
        # ">>> Object detection >>>"
        # ">>> Ultrasonic Sensors Detect >>>"
      }
      frame True {
        # ">> Item Selection Bias >>"
        # ">>> IR Sensors >>>"
        # ">>> Line Sensor Cluster>>>"
        # ">>> Line Sensor Cluster>>>"
        # ">>> Motor control cluster >>>"
        # ">>> yStepper command>>>"
        # ">>> IR Sensors >>>"
        # ">>> Motor control cluster >>>"
        # ">>State Logic Queue Reference >>"
        # ">>Timeout>>"
        # ">>> yStepper command>>>"
        # ">>> Time cluster >>>"
        # ">>> Object detection >>>"
        # ">>> Yaw >>>"
        # ">>> Ultrasonic Sensors Detect >>>"
        # ">>> Encoders >>>"
        # ">>> Stepper position >>>"
        # ">>State Logic  >>"
        # ">>True Stop Next State >>"
        # ">>Action Queue>>"
        # ">> Manual override >>"
        # ">>> Time cluster >>>"
        # ">>> Yaw >>>"
        # ">>> Stepper position >>>"
        # ">>> Encoders >>>"
        # ">>> Object detection >>>"
        # ">>> Ultrasonic Sensors Detect >>>"
        # ">>Action Queue>>"
        # ">>State Logic Queue Reference >>"
        n187 = Or(x=w313, y=w314) -> (x .or. y?=w312:bool)
        n188 = Unbundle By Name(w293) -> ("Left IR Sensor"=w294:dbl, "Arm IR Sensor"=w290:dbl, "Bottom IR Sensor"=w285:dbl)
        n189 = Unbundle By Name(w288) -> ("Line Detected?"=w289:bool)
        n190 = Unbundle By Name(w299) -> ("Time up flag"=w300:bool)
        n191 = Unbundle By Name(w301) -> ("Yaw"=w302:dbl, "Compass"=w296:dbl)
        n192 = Unbundle By Name(w303) -> ("y Stepper Position"=w305:u8, "z Stepper Position"=w304:u8)
        n193 = Unbundle By Name(w319) -> ("xDistance"=w316:dbl, "yDistance"=w317:dbl, "wDistance"=w318:dbl)
        n194 = Unbundle By Name(w307) -> ("Recognized Object"=w306:bool, "Object X coordinate"=w309:dbl, "Object Y coordinate"=w308:dbl)
        n195 = Unbundle By Name(w330) -> ("PING_A"=w322:u8, "PING_B"=w321:u8, "PING_C"=w320:u8, "PING_D"=w315:u8)
        n196 = case shown="1" w329 {
          tunnel: [w335 w347 w361 w372 w490 w507 w553 w590 w645 w687 w735 w779 w834 w882 w926 w986 w1027 w1070 w1119 w1162 w1215 w1253 w1305 w1349 w1393 w1423 w1441 w1487 w1528 w1577 w1630 w1669 w1718 w1761 w1814 w1852 w1904 w1940 w1989 w2032 w2082 w2126 w2171 w2223 w2264 w2312 w2351 w2393 w2448 w2502 w2540 w2586 w2635 w2676 w2720] -> w328
          tunnel: w327 -> [w335 w350 w362 w375 w492 w508 w554 w599 w643 w691 w736 w785 w827 w885 w933 w976 w1030 w1076 w1118 w1165 w1205 w1259 w1295 w1344 w1384 w1423 w1431 w1490 w1534 w1576 w1629 w1675 w1717 w1764 w1804 w1858 w1894 w1944 w1996 w2037 w2087 w2131 w2175 w2221 w2265 w2313 w2353 w2403 w2458 w2501 w2544 w2592 w2634 w2680 w2724]
          tunnel: [State_Type_Definitions,_for_0.26g_versions_and_later_2."Idle" ("Enum") State_Type_Definitions,_for_0.26g_versions_and_later_2."Idle" ("Enum") w357 w374 State_Type_Definitions,_for_0.26g_versions_and_later_2."Shutdown" ("Enum") w509 w555 w597 w646 w688 w734 w780 w833 w883 w928 w985 w1028 w1077 w1120 w1164 w1214 w1260 w1304 w1350 w1385 State_Type_Definitions,_for_0.26g_versions_and_later_2."Idle" ("Enum") w1440 w1488 w1535 w1578 w1631 w1676 w1719 w1763 w1813 w1859 w1903 w1941 w1990 w2033 w2083 w2127 w2172 w2224 w2263 w2311 w2352 w2398 w2459 w2503 w2541 w2587 w2636 w2677 w2721] -> w326
          tunnel: w325 -> [_ _ w360 w378 _ w513 w560 w593 w642 w692 w743 w784 w831 w886 w932 w983 w1025 w1075 w1116 w1166 w1212 w1258 w1302 w1347 w1392 _ w1438 w1485 w1533 w1574 w1627 w1674 w1715 w1765 w1811 w1857 w1901 w1948 w1995 w2040 w2090 w2134 w2178 w2220 w2266 w2306 w2354 w2402 w2457 w2500 w2548 w2591 w2633 w2684 w2725]
          tunnel: w324 -> [_ _ _ w377 _ w512 w559 w592 w641 w693 w742 w783 w830 w879 w931 w982 w1024 w1074 w1115 w1167 w1211 w1257 w1301 w1346 w1390 _ w1437 w1484 w1532 w1573 w1626 w1673 w1714 w1766 w1810 w1856 w1900 w1943 w1994 w2039 w2089 w2133 w2174 w2219 w2267 w2307 w2355 w2401 w2456 w2499 w2547 w2590 w2632 w2683 w2726]
          tunnel: w323 -> [_ _ w359 w373 _ w511 w558 w591 w640 w694 w741 w782 w829 w878 w930 w984 w1026 w1073 w1114 w1168 w1213 w1256 w1303 w1345 w1391 _ w1439 w1486 w1531 w1572 w1625 w1672 w1713 w1767 w1812 w1855 w1902 w1947 w1993 w2038 w2088 w2132 w2177 w2218 w2268 w2308 w2356 w2400 w2455 w2498 w2546 w2589 w2631 w2682 w2727]
          tunnel: w312 -> [_ _ _ _ _ w498 w552 w598 w639 w695 w738 w778 w832 w884 w934 w977 w1031 w1071 w1117 w1169 w1206 w1254 w1296 w1348 w1388 _ w1432 w1491 w1529 w1575 w1628 w1670 w1716 w1768 w1805 w1853 w1895 w1946 w1988 w2036 w2086 w2130 w2176 w2217 w2269 w2309 w2357 w2399 w2454 w2497 w2545 w2588 w2630 w2681 w2728]
          tunnel: w322 -> [_ _ _ _ _ _ _ _ _ _ _ _ _ _ _ _ _ _ _ _ _ _ _ _ _ _ _ _ _ _ _ _ _ _ _ _ _ _ _ _ _ _ _ _ _ _ _ _ _ _ _ _ _ _ _]
          tunnel: w321 -> [_ _ _ _ _ _ _ _ w638 _ _ _ w823 w867 w924 _ _ _ _ _ _ _ _ _ _ _ _ w1477 _ _ _ _ _ _ _ _ _ _ _ _ _ _ _ _ _ _ _ _ w2452 _ _ _ _ _ _]
          tunnel: w320 -> [_ _ _ _ _ _ _ _ w637 _ _ _ w824 w868 w925 _ _ _ _ _ _ _ _ _ _ _ _ w1478 _ _ _ _ _ _ _ _ _ _ _ _ _ _ _ _ _ _ _ _ w2453 _ _ _ _ _ _]
          tunnel: w318 -> [_ _ _ _ _ _ _ _ _ _ w740 _ _ _ _ _ _ _ _ _ _ _ _ _ _ _ _ _ _ _ _ _ _ _ _ _ _ _ _ _ _ _ _ _ _ _ _ w2396 _ _ _ _ _ _ _]
          tunnel: w317 -> [_ _ _ _ _ w506 w551 _ _ w686 _ _ _ _ w929 _ _ _ _ _ _ _ _ _ _ _ _ _ _ _ _ _ _ _ _ _ _ _ _ _ _ _ _ _ _ _ _ _ w2444 _ _ _ _ _ _]
          tunnel: w316 -> [_ _ _ _ _ _ _ _ _ _ _ _ _ w873 _ _ _ _ _ _ _ _ _ _ _ _ _ _ _ _ w1616 _ _ _ _ _ _ _ _ _ _ _ _ _ w2258 _ _ _ _ _ _ _ w2629 _ _]
          tunnel: w315 -> [_ _ _ _ _ _ _ _ _ _ _ _ _ _ _ _ _ _ _ _ _ _ _ _ _ _ _ _ _ _ _ _ _ _ _ _ _ _ _ _ _ _ _ _ _ _ _ _ _ _ _ _ _ _ _]
          tunnel: [State_Type_Definitions,_for_0.26g_versions_and_later_2."Idle" ("Enum") State_Type_Definitions,_for_0.26g_versions_and_later_2."Idle" ("Enum") State_Type_Definitions,_for_0.26g_versions_and_later_2."Idle" ("Enum") State_Type_Definitions,_for_0.26g_versions_and_later_2."Idle" ("Enum") State_Type_Definitions,_for_0.26g_versions_and_later_2."Shutdown" ("Enum") w504 w549 w596 w644 w689 w731 w777 w826 w881 w927 w987 w1029 w1069 w1121 w1163 w1216 w1252 w1306 w1351 w1386 w1425 w1442 w1489 w1527 w1579 w1632 w1668 w1720 w1762 w1815 w1851 w1905 w1942 w1991 w2035 w2085 w2129 w2173 w2222 w2262 w2310 w2350 w2397 w2460 w2504 w2542 w2585 w2637 w2678 w2722] -> w311
          tunnel: w310 -> [_ _ w357 _ _ _ _ _ _ _ _ _ _ _ _ _ _ _ _ _ _ _ _ _ _ w1425 _ _ _ _ _ _ _ _ _ _ _ _ _ _ _ _ _ _ _ _ _ _ _ _ _ _ _ _ _]
          tunnel: w306 -> [_ _ _ _ _ _ _ _ _ _ _ _ _ _ _ _ _ _ _ _ _ _ _ _ w1387 _ _ _ _ _ _ _ _ _ _ _ _ _ _ _ _ _ _ _ _ _ _ _ _ _ _ _ _ _ _]
          tunnel: w309 -> [_ _ _ _ _ _ _ _ _ _ _ _ _ _ _ _ _ _ _ _ _ _ _ _ _ _ _ _ _ _ w1622 _ _ _ _ _ _ _ _ _ _ _ _ _ _ _ _ _ _ _ _ _ _ _ _]
          tunnel: w308 -> [_ _ _ _ _ _ _ _ _ _ _ _ _ _ _ _ _ _ _ w1158 _ _ _ _ _ _ _ _ _ _ _ _ _ w1757 _ _ _ _ _ _ _ _ _ _ _ _ _ _ _ _ _ _ _ _ _]
          tunnel: w305 -> [_ _ _ _ _ _ _ _ _ _ _ _ _ _ _ _ _ _ _ w1157 _ _ _ _ _ _ _ _ _ _ _ _ _ w1756 _ _ _ _ _ _ _ _ _ _ _ _ _ _ _ _ _ _ _ _ _]
          tunnel: w304 -> [_ _ _ _ _ _ _ w595 _ _ _ w775 _ _ _ w980 _ w1065 _ _ w1209 _ w1299 w1343 _ _ w1435 _ _ _ _ _ _ _ w1808 _ w1898 w1945 _ _ _ _ _ _ _ _ _ _ _ _ _ _ _ _ _]
          tunnel: w302 -> [_ _ _ _ _ _ _ _ _ _ _ _ _ _ _ _ _ _ _ _ _ _ _ _ _ _ _ _ _ _ _ _ _ _ _ _ _ _ _ _ _ _ _ _ _ _ _ _ _ _ _ _ _ _ _]
          tunnel: w300 -> [_ _ _ _ _ _ _ _ _ _ _ _ _ _ _ _ w1019 _ w1111 _ _ w1250 _ _ _ _ _ _ w1525 w1569 _ w1666 w1710 _ _ w1849 _ _ _ _ _ _ w2167 _ _ w2305 w2349 _ _ _ w2543 w2584 _ w2679 w2723]
          tunnel: w298 -> [w333 w345 w356 w370 w488 w503 w548 w594 w636 w690 w730 w776 w825 w877 w923 w975 w1022 w1068 w1112 w1160 w1204 w1251 w1294 w1340 w1383 w1426 w1430 w1482 w1526 w1570 w1623 w1667 w1711 w1759 w1803 w1850 w1893 w1939 w1992 w2034 w2084 w2128 w2170 w2216 w2271 w2315 w2359 w2405 w2462 w2506 w2550 w2594 w2642 w2686 w2730]
          tunnel: [w333 w344 w356 w370 w488 w503 w548 w594 w636 w690 w730 w776 w825 w877 w923 w975 w1022 w1068 w1112 w1159 w1204 w1251 w1294 w1340 w1383 w1426 w1430 w1482 w1526 w1570 w1623 w1667 w1711 w1758 w1803 w1850 w1893 w1939 w1992 w2034 w2084 w2128 w2170 w2216 w2271 w2315 w2359 w2405 w2462 w2506 w2550 w2594 w2642 w2686 w2730] -> w297
          tunnel: w296 -> [_ _ _ _ _ _ _ _ _ _ _ _ _ _ _ _ _ _ _ _ _ _ _ _ _ _ _ _ _ _ _ _ _ _ _ _ _ _ w1987 _ _ _ _ _ _ _ _ _ _ _ _ _ _ _ _]
          tunnel: [_ _ _ TRUE _ _ _ _ _ _ _ _ _ _ _ _ _ _ _ _ _ _ _ _ _ _ _ _ _ _ _ _ _ _ _ _ _ _ _ _ _ _ _ _ _ _ _ _ _ _ _ _ _ _ _] -> w295
          tunnel: w294 -> [_ _ _ _ _ _ _ _ _ _ _ _ _ _ _ _ _ _ _ _ _ _ _ _ _ _ _ _ _ _ _ _ _ _ _ _ _ _ _ _ _ _ _ _ _ _ _ _ _ _ _ _ _ _ _]
          tunnel: w292 -> [w332 w342 w355 w368 w487 w502 w547 w589 w635 w683 w729 w772 w818 w866 w922 w974 w1021 w1067 w1110 w1154 w1203 w1249 w1293 w1339 w1382 w1427 w1429 w1475 w1524 w1568 w1619 w1665 w1709 w1753 w1802 w1848 w1892 w1938 w1983 w2031 w2081 w2125 w2169 w2215 w2273 w2317 w2361 w2407 w2464 w2508 w2552 w2596 w2644 w2688 w2732]
          tunnel: [w332 w341 w355 w368 w487 w502 w547 w589 w635 w683 w729 w772 w818 w866 w922 w974 w1021 w1067 w1110 w1154 w1203 w1249 w1293 w1339 w1382 w1427 w1429 w1475 w1524 w1568 w1618 w1665 w1709 w1753 w1802 w1848 w1892 w1938 w1983 w2031 w2081 w2125 w2169 w2215 w2273 w2317 w2361 w2407 w2464 w2508 w2552 w2596 w2644 w2688 w2732] -> w291
          tunnel: w290 -> [_ _ _ _ _ _ _ _ _ _ _ _ _ _ _ _ _ _ _ _ _ _ _ _ _ _ _ _ _ _ _ _ _ _ _ _ _ _ _ _ w2079 _ _ w2214 _ _ _ _ w2450 _ _ _ _ _ _]
          tunnel: w289 -> [_ _ _ _ _ w499 _ _ _ _ _ _ _ _ w920 _ _ _ _ _ _ _ _ _ _ _ _ _ _ _ _ _ _ _ _ _ _ _ _ w2030 _ w2123 _ _ w2260 _ _ _ _ w2496 _ _ w2628 _ _]
          tunnel: [w331 w337 w354 w367 w486 w501 w546 w588 w634 w682 w728 w771 w817 w865 w921 w973 w1020 w1066 w1109 w1153 w1202 w1248 w1292 w1338 w1381 w1422 w1428 w1474 w1523 w1567 w1611 w1664 w1708 w1752 w1801 w1847 w1891 w1937 w1982 w2029 w2078 w2124 w2168 w2211 w2272 w2316 w2360 w2406 w2463 w2507 w2551 w2595 w2643 w2687 w2731] -> w287
          tunnel: w286 -> [w331 w337 w354 _ w486 w501 w546 w588 w634 w682 w728 w771 w817 w865 w921 w973 w1020 w1066 w1109 w1153 w1202 w1248 w1292 w1338 w1381 w1422 w1428 w1474 w1523 w1567 w1611 w1664 w1708 w1752 w1801 w1847 w1891 w1937 w1982 w2029 w2078 w2124 w2168 w2211 w2272 w2316 w2360 w2406 w2463 w2507 w2551 w2595 w2643 w2687 w2731]